vi "Main.vi"() -> ()   [LabVIEW 2015] (continued)
        n125 = call <vilib>:"Check if File or Folder Exists.vi"("error in (no error)"=w361, "path"=w363) -> ("error out"=w365:errorcluster, "file or folder exists?"=w364:bool, "dup path"=w366:path)  [unwired: 7 in]
        n126 = case shown="False" w364 {
          tunnel: w365 -> [w370 w371]
          tunnel: [w369 w371] -> w356
          tunnel: [w368 w372] -> w351
          tunnel: w366 -> [w367 w372]
          frame False {
            n127 = Create Folder(path (use dialog)=w367, error in=w370) -> (created path=w368:path, error out=w369:errorcluster)  [unwired: 1 in, 1 out]
          }
          frame True {
          }
        }
        n128 = property on="Calibration AI  Signals (Integrated)" class="WFChart (strict)"() -> ("History Data"=w358:dbl[][])  [unwired: 2 in, 2 out]
        n129 = Index Array(array=w337, index=2) -> (element=w347:cluster{"X":dbl[], "Y":dbl[]})
        n130 = Index Array(array=w337, index=3) -> (element=w346:cluster{"X":dbl[], "Y":dbl[]})
        n131 = Index Array(array=w337, index=0) -> (element=w349:cluster{"X":dbl[], "Y":dbl[]})
        n132 = Index Array(array=w337, index=1) -> (element=w348:cluster{"X":dbl[], "Y":dbl[]})
        n133 = Unbundle By Name(w346) -> ("Y"=w341:dbl[])
        n134 = Unbundle(w349) -> ("X"=w345:dbl[], "Y"=w344:dbl[])
        n135 = Unbundle By Name(w348) -> ("Y"=w343:dbl[])
        n136 = Unbundle By Name(w347) -> ("Y"=w342:dbl[])
        n137 = Transpose 2D Array(2D array=w358) -> (transposed array=w357:dbl[][])
        n138 = Build Array(w345, w344, w343, w342, w341) -> (w340:dbl[][])
        n139 = Transpose 2D Array(2D array=w340) -> (transposed array=w339:dbl[][])
        n140 = call "Save2CSV.vi"("Time Stamp?"=FALSE, "File Name"=w329, "error in"=w356, "Data Name"="Raw" ("string"), "Data 2D Array"=w357, "Parent Directory"=w351) -> ("error out"=w352:errorcluster)  [unwired: 4 in, 1 out]
        n141 = call "Save2CSV.vi"("Time Stamp?"=FALSE, "File Name"=w329, "error in"=w352, "Data Name"="Phase" ("string"), "Data 2D Array"=w339, "Parent Directory"=w351) -> ("error out"=w338:errorcluster)  [unwired: 4 in, 1 out]
      }
      event "Save #1": Value Change {
        n142 = event-data() -> ()  [unwired: 1 in, 1 out]
        n143 = local read "Wavelength (nm)"() -> (w380:string)
        n144 = local write "Wavelength #1"(w380) -> ()
        "[M/B]#1" <- "[M/B]"
        "Calibrated Bias #1" <- "Calibrated Bias (V)"
        "[O_B] #1" <- "[O_B]"
        "[d13]#1" <- "[d13]"
        "[d24]#1" <- "[d24]"
      }
      event "Load #1": Value Change {
        n145 = event-data() -> ()  [unwired: 1 in, 1 out]
        n146 = local read "[O_B] #1"() -> (w388:dbl)
        n147 = local read "[d13]#1"() -> (w384:dbl)
        n148 = local read "[d24]#1"() -> (w383:dbl)
        n149 = local read "Calibrated Bias #1"() -> (w390:dbl[])
        n150 = local read "[M/B]#1"() -> (w389:dbl)
        n151 = local write "[O_B]"(w388) -> ()
        n152 = local write "Calibrated Bias (V)"(w390) -> ()
        n153 = local write "Wavelength (nm)"("Wavelength #1") -> ()
        n154 = local write "[M/B]"(w389) -> ()
        n155 = local write "[d13]"(w384) -> ()
        n156 = local write "[d24]"(w383) -> ()
      }
      event "Save #2": Value Change {
        n157 = event-data() -> ()  [unwired: 1 in, 1 out]
        n158 = local read "[d13]"() -> (→"[d13]#2":dbl)
        n159 = local read "[O_B]"() -> (→"[O_B]#2":dbl)
        n160 = local read "[d24]"() -> (→"[d24]#2":dbl)
        n161 = local read "Calibrated Bias (V)"() -> (→"Calibrated Bias #2":dbl[])
        n162 = local read "Wavelength (nm)"() -> (w397:string)
        n163 = local read "[M/B]"() -> (→"[M/B]#2":dbl)
        n164 = local write "Wavelength #2"(w397) -> ()
      }
      event "Load #2": Value Change {
        n165 = event-data() -> ()  [unwired: 1 in, 1 out]
        n166 = local read "[O_B]#2"() -> (w408:dbl)
        n167 = local read "[d13]#2"() -> (w404:dbl)
        n168 = local read "Calibrated Bias #2"() -> (w412:dbl[])
        n169 = local read "[d24]#2"() -> (w403:dbl)
        n170 = local read "[M/B]#2"() -> (w411:dbl)
        n171 = local write "[O_B]"(w408) -> ()
        n172 = local write "Wavelength (nm)"("Wavelength #2") -> ()
        n173 = local write "Calibrated Bias (V)"(w412) -> ()
        n174 = local write "[M/B]"(w411) -> ()
        n175 = local write "[d24]"(w403) -> ()
        n176 = local write "[d13]"(w404) -> ()
      }
      event "Save #3": Value Change {
        n177 = event-data() -> ()  [unwired: 1 in, 1 out]
        n178 = local read "[O_B]"() -> (→"[O_B]#3":dbl)
        n179 = local read "[d24]"() -> (→"[d24]#3":dbl)
        n180 = local read "[d13]"() -> (→"[d13]#3":dbl)
        n181 = local read "Calibrated Bias (V)"() -> (→"Calibrated Bias #3":dbl[])
        n182 = local read "Wavelength (nm)"() -> (w417:string)
        n183 = local read "[M/B]"() -> (→"[M/B]#3":dbl)
        n184 = local write "Wavelength #3"(w417) -> ()
      }
      event "Load #3": Value Change {
        n185 = event-data() -> ()  [unwired: 1 in, 1 out]
        n186 = local read "[O_B]#3"() -> (w428:dbl)
        n187 = local read "[d13]#3"() -> (w424:dbl)
        n188 = local read "[d24]#3"() -> (w423:dbl)
        n189 = local read "Calibrated Bias #3"() -> (w430:dbl[])
        n190 = local read "[M/B]#3"() -> (w429:dbl)
        n191 = local write "[O_B]"(w428) -> ()
        n192 = local write "Wavelength (nm)"("Wavelength #3") -> ()
        n193 = local write "Calibrated Bias (V)"(w430) -> ()
        n194 = local write "[M/B]"(w429) -> ()
        n195 = local write "[d13]"(w424) -> ()
        n196 = local write "[d24]"(w423) -> ()
      }
      event "Save #4": Value Change {
        n197 = event-data() -> ()  [unwired: 1 in, 1 out]
        n198 = local read "[d13]"() -> (→"[d13]#4":dbl)
        n199 = local read "[d24]"() -> (→"[d24]#4":dbl)
        n200 = local read "[O_B]"() -> (→"[O_B]#4":dbl)
        n201 = local read "Calibrated Bias (V)"() -> (→"Calibrated Bias #4":dbl[])
        n202 = local read "Wavelength (nm)"() -> (w437:string)
        n203 = local read "[M/B]"() -> (→"[M/B]#4":dbl)
        n204 = local write "Wavelength #4"(w437) -> ()
      }
      event "Load #4": Value Change {
        n205 = event-data() -> ()  [unwired: 1 in, 1 out]
        n206 = local read "[O_B]#4"() -> (w448:dbl)
        n207 = local read "[d13]#4"() -> (w444:dbl)
        n208 = local read "Calibrated Bias #4"() -> (w450:dbl[])
        n209 = local read "[d24]#4"() -> (w443:dbl)
        n210 = local read "[M/B]#4"() -> (w449:dbl)
        n211 = local write "[O_B]"(w448) -> ()
        n212 = local write "Wavelength (nm)"("Wavelength #4") -> ()
        n213 = local write "Calibrated Bias (V)"(w450) -> ()
        n214 = local write "[M/B]"(w449) -> ()
        n215 = local write "[d13]"(w444) -> ()
        n216 = local write "[d24]"(w443) -> ()
      }
      event "Fast Scan": Value Change {
        # "Repeat for Fast Scan"
        n217 = event-data() -> ()  [unwired: 1 in, 1 out]
        n218 = flat-sequence {
          tunnel: w469 -> [w476]
          tunnel: [w476] -> w465
          tunnel: [w475] -> w464
          tunnel: [w474] -> w463
          tunnel: w467 -> [w474]
          tunnel: [w473] -> w462
          tunnel: w466 -> [w473]
          tunnel: w461 -> [w471]
          tunnel: [w470] -> w460
          tunnel: w465 -> [w502]
          tunnel: [w502] -> w457
          tunnel: w464 -> [w501]
          tunnel: [w501] -> w456
          tunnel: w463 -> [w497]
          tunnel: w462 -> [w484]
          tunnel: [w494] -> w455
          tunnel: w460 -> [w493]
          tunnel: [w482] -> w453
          tunnel: [w529] -> w459
          tunnel: [w530] -> w468
          tunnel: w457 -> [w530]
          tunnel: w455 -> [w526]
          tunnel: w456 -> [w520]
          tunnel: w453 -> [w513]
          frame #0 {
            n219 = local read "Shutter"() -> (w472:bool)
            n220 = case shown="False" w472 {
              tunnel: w471 -> [w479 w481]
              tunnel: [w478 w481] -> w470
              frame False {
                n221 = call "ShutterControl.vi"("error in"=w479, "Shutter"=TRUE) -> ("error out"=w478:errorcluster, "Status Indicator"=w477:bool)  [unwired: 8 in]
                n222 = local write "Shutter"(w477) -> ()
              }
              frame True {
              }
            }
            n223 = Tick Count (ms)() -> (millisecond timer value=w475:u32)
          }
          frame #1 {
            w487 = T13."Fast Scan" ("Main Tab")
            n224 = call "DAQInit.vi"("Scan/Meas Parameters"="Fast Scan Parameters", "error in"=w493, "Functions"=w487, "Global Parameters"=w484, "DAQ Channels"=w497) -> ("error out"=w495:errorcluster, "Expected Time (s)"=→"Expected Frame Time (s)":dbl, "Tasks Out"=w499:T14)  [unwired: 4 in]
            n225 = call "ScanXY.vi"("Scan/Meas Parameters"="Fast Scan Parameters") -> ("XYcoordinates"=w488:dbl[][])  [unwired: 10 in]
            n226 = Unbundle By Name("Fast Scan Parameters") -> ("Pixel Size"=w492:dbl)
            n227 = case shown="True" "Single Pixel?" {
              tunnel: [w503 w504] -> w489
              tunnel: w488 -> [w503 w505]
              frame False {
              }
              frame True {
                n228 = Multiply(x=w505, y=0.0) -> (x*y=w504:dbl[][])
              }
            }
            n229 = To Long Integer(number=w492) -> (32bit integer=w491:i32)
            n230 = call "ImageFrame.vi"("Tasks In"=w499, "Functions"=w487, "error in"=w495, "XYcoordinates"=w489) -> ("Tasks Out"=w496:T14, "DC AI Channel Date"=w485:dbl[], "error out"=w498:errorcluster)  [unwired: 7 in, 2 out]
            n231 = call "Analysis.vi"("Functions"=w487, "Scan/Meas Parameters"="Fast Scan Parameters", "Global Parameters"=w484, "DC AI Channel Data"=w485) -> ("AI DC Data"=w482:dbl[])  [unwired: 2 in, 5 out]
            n232 = Reshape Array(w482, w491, w491) -> (→"Fast Scan Intensity Image":dbl[][])
            n233 = call "DAQClose.vi"("error in"=w498, "Functions"=w487, "Tasks In"=w496, "DAQ Channels"=w497) -> ("error out"=w494:errorcluster)  [unwired: 7 in]
          }
          frame #2 {
            n234 = local read "Simple Max Search"() -> (w516:bool)
            n235 = local read "Export Z Calibration"() -> (w507:bool)
            n236 = Tick Count (ms)() -> (millisecond timer value=w521:u32)
            n237 = call "ShutterControl.vi"("error in"=w526, "Shutter"=FALSE) -> ("error out"=w525:errorcluster, "Status Indicator"=w527:bool)  [unwired: 8 in]
            n238 = local read "Quadratic Search"() -> (w509:bool)
            n239 = local write "Shutter"(w527) -> ()
            n240 = call <vilib>:"Std Deviation and Variance.vi"("X"=w513) -> ("mean"=w508:dbl, "variance"=w514:dbl)  [unwired: 1 in, 1 out]
            "Mean Pixel Value" <- w508
            n241 = Subtract(x=w521, y=w520) -> (x-y=w523:u32)
            n242 = Square(x=w508) -> (x^2=w515:dbl)
            n243 = local read "SPGD"() -> (w517:bool)
            n244 = To Double Precision Float(number=w523) -> (double precision float=w524:dbl)
            n245 = Divide(x=w514, y=w515) -> (x/y=w510:dbl)
            "Normalized Variance" <- w510
            n246 = Divide(x=w524, y=1000.0) -> (x/y=→"Actual Scan Time (s)":dbl)
            n247 = Compound Arithmetic op=OR(w509, w517, w516, w507) -> (w518:bool)
            n248 = case shown="False" w518 {
              tunnel: [w546 w553] -> w529
              tunnel: w525 -> [w544 w553]
              frame False {
                n249 = local read "Fast Scan Progress"() -> (w540:dbl)
                n250 = Reciprocal(x="Fast Scan Frames") -> (1/x=w541:dbl)
                n251 = Multiply(x=100.0, y=w541) -> (x*y=w543:dbl)
                n252 = Add(x=w540, y=w543) -> (x+y=w536:dbl)
                "Fast Scan Progress" <- w536
                n253 = Greater Or Equal?(x=w536, y=100.0) -> (x >= y?=w537:bool)
                n254 = Compound Arithmetic op=OR(w537, "Stop Fast Scan") -> (w545:bool)
                n255 = case shown="True" w545 {
                  tunnel: w544 -> [w549 w550]
                  tunnel: [w548 w550] -> w546
                  frame False {
                    # "Continue Fast Scan"
                    n256 = property on="Fast Scan" class="Bool (strict)"(error in=w549, "Val(Sgnl)"=TRUE ("Value (Signaling)")) -> (error out=w548:errorcluster)  [unwired: 1 in, 1 out]
                  }
                  frame True {
                    w552 = FALSE ("Fast Scan")
                    # "Fast Scan Stops"
                    n257 = local write "Fast Scan Progress"(0.0 ("Fast Scan Progress")) -> ()
                    n258 = local write "Fast Scan"(w552) -> ()
                    n259 = local write "Stop Fast Scan"(w552) -> ()
                  }
                }
              }
              frame True {
              }
            }
            n260 = case shown="\"Mean Squared Pixel Value\"" "Optimization Metric" {
              tunnel: [w531 w532 w533] -> w511
              tunnel: w508 -> [w531 _ w534]
              tunnel: w510 -> [_ w532 _]
              frame "Mean Pixel Value", Default {
              }
              frame "Normalized Variance" {
              }
              frame "Mean Squared Pixel Value" {
                n261 = Square Root(x=w534) -> (sqrt(x)=w533:dbl)
              }
            }
            "Metric Value" <- w511
          }
        }
      }
      event "Relax DM": Value Change {
        w566 = u32 0 items=["Mirror", "Arms", "Mirror + Arms"] ("Device Part (Mirror)")
        # "First Step"
        n262 = event-data() -> ()  [unwired: 1 in, 1 out]
        n263 = call "TLDFMX Relax.vi"("Reload (1)"=TRUE, "error in (no error)"=w554, "Is First Step (0)"=TRUE, "Device Part (Mirror)"=w566, "instrument handle"=w555) -> ("error out"=w562:errorcluster, "Relax Pattern Mirror (0)"=w561:dbl[], "instrument handle out"=w563:refnum<visa-resource-name>)  [unwired: 2 in, 2 out]
        n264 = call "TLDFM Set Segment Voltages.vi"("error in (no error)"=w562, "Segment Voltages"=w561, "instrument handle"=w563) -> ("error out"=w559:errorcluster, "instrument handle out"=w560:refnum<visa-resource-name>)  [unwired: 7 in]
        n265 = while {
          tunnel: w560 -> [w573]
          tunnel: w559 -> [w572]
          tunnel: [w569] -> w558
          tunnel: [w568] -> w557
          stop <- w570 stop-if-true
          w574 = u32 0 items=["Mirror", "Arms", "Mirror + Arms"] ("Device Part (Mirror)")
          # "Loop Until Remaining Relax Steps Are 0"
          n266 = call "TLDFMX Relax.vi"("Reload (1)"=TRUE, "error in (no error)"=w572, "Is First Step (0)"=FALSE, "Device Part (Mirror)"=w574, "instrument handle"=w573) -> ("error out"=w578:errorcluster, "Relax Pattern Mirror (0)"=w579:dbl[], "instrument handle out"=w577:refnum<visa-resource-name>, "Remaining Steps"=w571:i32)  [unwired: 2 in, 1 out]
          n267 = Less Or Equal To 0?(x=w571) -> (x <= 0?=w570:bool)
          n268 = call "TLDFM Set Segment Voltages.vi"("error in (no error)"=w578, "Segment Voltages"=w579, "instrument handle"=w577) -> ("error out"=w568:errorcluster, "instrument handle out"=w569:refnum<visa-resource-name>)  [unwired: 7 in]
        }
      }
      event "Reset Zernike": Value Change {
        n269 = event-data() -> ()  [unwired: 1 in, 1 out]
        n270 = call "TLDFMX Reset.vi"("error in (no error)"=w582, "instrument handle"=w583) -> ("error out"=w580:errorcluster, "instrument handle out"=w581:refnum<visa-resource-name>)  [unwired: 8 in]
        n271 = local write "Zernike Array"(dbl[] [0.0, 0.0, 0.0, 0.0, 0.0, 0.0, 0.0, 0.0, 0.0, 0.0, 0.0, 0.0] ("Zernike Array")) -> ()
      }
      event "Zernike Array", "Apply Zernike": Value Change {
        n272 = event-data() -> ()  [unwired: 1 in, 1 out]
        n273 = local read "Zernike Enable"() -> (w589:bool[])
        n274 = Boolean To (0,1)(Boolean=w589) -> (0, 1=w588:i16[])
        n275 = Multiply(x="Zernike Array", y=w588) -> (x*y=w586:dbl[])
        n276 = call "TLDFMX Calculate Zernike Pattern.vi"("error in (no error)"=w599, "Zernike Amplitudes"=w586, "Zernikes"=u32 4294967295, "instrument handle"=w597) -> ("error out"=w594:errorcluster, "Mirror Pattern"=w595:dbl[], "instrument handle out"=w596:refnum<visa-resource-name>)  [unwired: 5 in]
        n277 = call "TLDFM Set Segment Voltages.vi"("error in (no error)"=w594, "Segment Voltages"=w595, "instrument handle"=w596) -> ("error out"=w593:errorcluster, "instrument handle out"=w591:refnum<visa-resource-name>)  [unwired: 7 in]
      }
      event "Save Zernike": Value Change {
        w617 = "DM" ("section")
        n278 = event-data() -> ()  [unwired: 1 in, 1 out]
        n279 = Current VI's Path() -> (path=w601:path)
        n280 = Strip Path(path=w601) -> (stripped path=w600:path)  [unwired: 1 out]
        n281 = Build Path(base path=w600, name or relative path=path "config.ini" ("default name")) -> (appended path=w627:path)
        n282 = local read "Zernike Array"() -> (w611:dbl[])
        n283 = call <vilib>:"Open Config Data.vi"("error in (no error)"=w626, "create file if necessary (T)"=TRUE, "configuration file path"=w627) -> ("error out"=w625:errorcluster, "refnum"=w623:T15)  [unwired: 6 in, 1 out]
        n284 = Array To Spreadsheet String(delimiter (Tab)=",", array=w611, 3:"%#g" ("format string")) -> (spreadsheet string=w615:string)
        n285 = Search and Replace String(input string=w615, search string="\r\n") -> (result string=w610:string)  [unwired: 6 in, 3 out]
        n286 = call-poly <vilib>:"Write Key.vi"("section"=w617, "error in (no error)"=w625, "value"=w610, "key"="Zernike Array", "refnum"=w623) -> ("error out"=w619:errorcluster, "refnum out"=w621:T15)  [unwired: 4 in, 1 out]
        n287 = local read "Zernike Enable"() -> (w604:bool[])
        n288 = for {
          tunnel: w604 -> [w632] mode=indexing
          tunnel: [w631] -> w605 mode=indexing
          n289 = Select(t="TRUE", s=w632, f="FALSE") -> (s? t:f=w631:string)
        }
        n290 = Array To Spreadsheet String(delimiter (Tab)=",", array=w605, 3:"%s" ("format string")) -> (spreadsheet string=w609:string)
        n291 = Search and Replace String(input string=w609, search string="\r\n") -> (result string=w603:string)  [unwired: 6 in, 3 out]
        n292 = call-poly <vilib>:"Write Key.vi"("section"=w617, "error in (no error)"=w619, "value"=w603, "key"="Zernike Enable", "refnum"=w621) -> ("error out"=w618:errorcluster, "refnum out"=w620:T15)  [unwired: 4 in, 1 out]
        n293 = call <vilib>:"Close Config Data.vi"("error in (no error)"=w618, "refnum"=w620) -> ("error out"=w624:errorcluster)  [unwired: 8 in, 1 out]
      }
      event "Load Zernike": Value Change {
        n294 = event-data() -> ()  [unwired: 1 in, 1 out]
        n295 = Current VI's Path() -> (path=w642:path)
        n296 = Strip Path(path=w642) -> (stripped path=w641:path)  [unwired: 1 out]
        n297 = Build Path(base path=w641, name or relative path=path "config.ini" ("default name")) -> (appended path=w639:path)
        n298 = call <vilib>:"Check if File or Folder Exists.vi"("error in (no error)"=w638, "path"=w639) -> ("error out"=w637:errorcluster, "file or folder exists?"=w635:bool, "dup path"=w636:path)  [unwired: 7 in]
        n299 = case shown="True" w635 {
          tunnel: [w646 w670] -> w640
          tunnel: w637 -> [w646 w648]
          tunnel: w636 -> [_ w647]
          frame False {
          }
          frame True {
            w650 = "DM" ("section")
            n300 = call <vilib>:"Open Config Data.vi"("error in (no error)"=w648, "create file if necessary (T)"=FALSE, "configuration file path"=w647) -> ("error out"=w663:errorcluster, "refnum"=w664:T15)  [unwired: 6 in, 1 out]
            n301 = call-poly <vilib>:"Read Key.vi"("section"=w650, "error in (no error)"=w663, "key"="Zernike Array", "refnum"=w664) -> ("error out"=w655:errorcluster, "value"=w666:string, "refnum out"=w653:T15)  [unwired: 4 in, 1 out]
            n302 = Spreadsheet String To Array(delimiter (Tab)=",", format string="%s", spreadsheet string=w666, array type (2D Dbl)=dbl[] []) -> (array=w662:dbl[])
            n303 = local write "Zernike Array"(w662) -> ()
            n304 = call-poly <vilib>:"Read Key.vi"("section"=w650, "error in (no error)"=w655, "key"="Zernike Enable", "refnum"=w653) -> ("error out"=w654:errorcluster, "value"=w658:string, "refnum out"=w652:T15)  [unwired: 4 in, 1 out]
            n305 = Spreadsheet String To Array(delimiter (Tab)=",", format string="%s", spreadsheet string=w658, array type (2D Dbl)=string[] []) -> (array=w656:string[])
            n306 = for {
              tunnel: "TRUE" -> [w674]
              tunnel: w656 -> [w673] mode=indexing
              tunnel: [w672] -> w649 mode=indexing
              n307 = Equal?(x=w673, y=w674) -> (x = y?=w672:bool)
            }
            n308 = local write "Zernike Enable"(w649) -> ()
            n309 = call <vilib>:"Close Config Data.vi"("error in (no error)"=w654, "refnum"=w652) -> ("error out"=w670:errorcluster)  [unwired: 8 in, 1 out]
          }
        }
      }
      event "Quadratic Search": Value Change {
        n310 = event-data() -> ()  [unwired: 1 in, 1 out]
        n311 = while {
          tunnel: [w776] -> w682
          tunnel: [w778] -> w686
          stop <- w779 stop-if-true
          n312 = local read "Zernike Enable"() -> (w777:bool[])
          n313 = local read "Current Z Idx"() -> (w782:i32)
          n314 = Index Array(array=w777, index=w782) -> (element=w783:bool)
          n315 = Array Size(array=w777) -> (size(s)=w781:i32)
          n316 = case shown="True" w783 {
            tunnel: w782 -> [w787 w789]
            tunnel: [w786 w789] -> w776
            tunnel: [FALSE ("2D Time-Lapse Measure") TRUE ("2D Time-Lapse Measure")] -> w780
            frame False {
              n317 = local write "Z Direction"(TRUE ("Zernike Dir")) -> ()
              n318 = Increment(x=w787) -> (x+1=w786:i32)
            }
            frame True {
            }
          }
          n319 = Greater?(x=w776, y=w781) -> (0:w778:bool)
          n320 = local write "Current Z Idx"(w776) -> ()
          n321 = Compound Arithmetic op=OR(w780, w778) -> (w779:bool)
        }
        n322 = local read "Current Iteration"() -> (w675:sgl)
        n323 = local read "Quadratic Calc"() -> (w678:bool)
        n324 = case shown="False" w678 {
          tunnel: w677 -> [w689 w693]
          tunnel: [w689 w693] -> w676
          tunnel: w675 -> [w688 _]
          frame False {
            n325 = Equal To 0?(x=w688) -> (x = 0?=w687:bool)
            n326 = case shown="True" w687 {
              frame False {
              }
              frame True {
                n327 = local read "Zernike Array"() -> (w690:dbl[])
                n328 = local write "Optimal Z Idx"(0 ("Optimal Z Idx")) -> ()
                n329 = local write "Optimal Zernike"(w690) -> ()
              }
            }
          }
          frame True {
            n330 = local read "Bias Amplitude"() -> (w702:dbl)
            n331 = local read "Optimal Zernike"() -> (w696:dbl[])
            n332 = local read "Initial Metric"() -> (w704:dbl)
            n333 = local read "Metric Value"() -> (w703:dbl)
            n334 = local read "Last Metric"() -> (w705:dbl)
            n335 = local read "Optimal Z Idx"() -> (w692:i32)
            n336 = call "QuadraticOptimization.vi"("Bias Amplitude"=w702, "Neg Metric"=w703, "Initial Metric"=w704, "Pos Metric"=w705) -> ("Opt Variable (compared to 0)"=w694:dbl)  [unwired: 7 in]
            n337 = Index Array(array=w696, index=w692) -> (element=w698:dbl)
            n338 = Add(x=w698, y=w694) -> (x+y=w699:dbl)
            n339 = In Range and Coerce(upper limit=1.0 ("y"), x=w699, lower limit=-1.0 ("y")) -> (coerced(x)=w697:dbl)  [unwired: 1 out]
            n340 = Replace Array Subset(array=w696, new element=w697, index=w692) -> (→"Optimal Zernike":dbl[])
          }
        }
        n341 = local read "Stop AO Algorithm"() -> (w685:bool)
        n342 = Compound Arithmetic op=OR(w686, w685) -> (w684:bool)
        n343 = case shown="False" w684 {
          tunnel: w676 -> [w717 w765]
          tunnel: [w712 w764] -> w683
          tunnel: w680 -> [w718 w762]
          tunnel: [w719 w763] -> w679
          tunnel: w675 -> [w709 _]
          tunnel: w682 -> [w714 _]
          frame False {
            w711 = TRUE ("Value (Signaling)")
            n344 = Equal To 0?(x=w709) -> (x = 0?=w715:bool)
            n345 = case shown="False" w715 {
              tunnel: [w738 w755] -> w710
              tunnel: [w740 w756] -> w706
              tunnel: w714 -> [w726 _]
              frame False {
                n346 = local read "Initial Zernike"() -> (w727:dbl[])
                n347 = local read "Z Direction"() -> (w737:bool)
                n348 = case shown="False" w737 {
                  tunnel: "Bias Amplitude" -> [w748 w753]
                  tunnel: [w747 w753] -> w735
                  tunnel: [FALSE ("Zernike Dir") TRUE ("Zernike Dir")] -> w730
                  tunnel: w726 -> [w744 _]
                  frame False {
                    # "Negative Bias"
                    n349 = Multiply(x=w748, y=-1.0) -> (x*y=w747:dbl)
                    "Quadratic Calc" <- TRUE ("Quadratic Calc")
                    "Optimal Z Idx" <- w744
                  }
                  frame True {
                    # "Positive Bias"
                    n350 = local write "Quadratic Calc"(FALSE ("Zernike Dir")) -> ()
                    n351 = local write "Z Direction"(FALSE ("Zernike Dir")) -> ()
                  }
                }
                n352 = Index Array(array=w727, index=w726) -> (element=w739:dbl)
                n353 = Add(x=w739, y=w735) -> (x+y=w732:dbl)
                n354 = In Range and Coerce(upper limit=1.0 ("y"), x=w732, lower limit=-1.0 ("y")) -> (coerced(x)=w731:dbl, In Range?=w729:bool)
                n355 = Compound Arithmetic op=AND(w729, w730) -> (w728:bool)
                n356 = case shown="False" w728 {
                  tunnel: w726 -> [w742 _]
                  frame False {
                    n357 = Increment(x=w742) -> (x+1=w743:i32)
                    n358 = local write "Z Direction"(TRUE ("Zernike Dir")) -> ()
                    n359 = local write "Current Z Idx"(w743) -> ()
                  }
                  frame True {
                  }
                }
                n360 = local read "Metric Value"() -> (w740:dbl)
                n361 = Replace Array Subset(array=w727, new element=w731, index=w726) -> (w738:dbl[])
              }
              frame True {
                n362 = local read "Zernike Array"() -> (w755:dbl[])
                "Initial Zernike" <- w755
                n363 = local read "Last Metric"() -> (w756:dbl)
                n364 = local write "Quadratic Calc"(FALSE ("Zernike Dir")) -> ()
              }
            }
            n365 = Increment(x=w709) -> (x+1=w716:sgl)
            n366 = local write "Current Iteration"(w716) -> ()
            n367 = call "TLDFMX Calculate Zernike Pattern.vi"("error in (no error)"=w717, "Zernike Amplitudes"=w710, "Zernikes"=u32 4294967295, "instrument handle"=w718) -> ("error out"=w721:errorcluster, "Mirror Pattern"=w722:dbl[], "instrument handle out"=w723:refnum<visa-resource-name>)  [unwired: 5 in]
            n368 = call "TLDFM Set Segment Voltages.vi"("error in (no error)"=w721, "Segment Voltages"=w722, "instrument handle"=w723) -> ("error out"=w720:errorcluster, "instrument handle out"=w719:refnum<visa-resource-name>)  [unwired: 7 in]
            n369 = Equal?(x=w709, y=sgl 1.0) -> (x = y?=w707:bool)
            n370 = property on="Fast Scan" class="Bool (strict)"(error in=w720, "Val(Sgnl)"=w711) -> (error out=w713:errorcluster)  [unwired: 1 in, 1 out]
            n371 = case shown="True" w707 {
              tunnel: w706 -> [_ w725]
              frame False {
              }
              frame True {
                "Initial Metric" <- w725
              }
            }
            n372 = local write "Zernike Array"(w710) -> ()
            n373 = property on="Quadratic Search" class="Bool (strict)"(error in=w713, "Val(Sgnl)"=w711) -> (error out=w712:errorcluster)  [unwired: 1 in, 1 out]
            n374 = local write "Last Metric"(w706) -> ()
          }
          frame True {
            w775 = FALSE ("2D Time-Lapse Measure")
            n375 = local read "Zernike Enable"() -> (w761:bool[])
            n376 = local read "Optimal Zernike"() -> (w759:dbl[])
            n377 = Boolean To (0,1)(Boolean=w761) -> (0, 1=w760:i16[])
            n378 = Multiply(x=w759, y=w760) -> (x*y=w758:dbl[])
            n379 = call "TLDFMX Calculate Zernike Pattern.vi"("error in (no error)"=w765, "Zernike Amplitudes"=w758, "Zernikes"=u32 4294967295, "instrument handle"=w762) -> ("error out"=w766:errorcluster, "Mirror Pattern"=w767:dbl[], "instrument handle out"=w768:refnum<visa-resource-name>)  [unwired: 5 in]
            n380 = local write "Zernike Array"(w759) -> ()
            n381 = call "TLDFM Set Segment Voltages.vi"("error in (no error)"=w766, "Segment Voltages"=w767, "instrument handle"=w768) -> ("error out"=w764:errorcluster, "instrument handle out"=w763:refnum<visa-resource-name>)  [unwired: 7 in]
            n382 = local write "Quadratic Calc"(FALSE ("Zernike Dir")) -> ()
            n383 = local write "Optimal Z Idx"(0 ("Optimal Z Idx")) -> ()
            n384 = local write "Current Iteration"(sgl 0.0 ("Current Step")) -> ()
            n385 = local write "Quadratic Search"(w775) -> ()
            n386 = local write "Z Direction"(TRUE ("Zernike Dir")) -> ()
            n387 = local write "Fast Scan Progress"(0.0 ("Fast Scan Progress")) -> ()
            n388 = local write "Current Z Idx"(0 ("Curr Zernike Idx")) -> ()
            n389 = local write "Fast Scan"(w775) -> ()
            n390 = local write "Stop Fast Scan"(w775) -> ()
            n391 = local write "Stop AO Algorithm"(w775) -> ()
          }
        }
      }
      event "Simple Max Search": Value Change {
        n392 = event-data() -> ()  [unwired: 1 in, 1 out]
        n393 = while {
          tunnel: [w800] -> w790
          tunnel: [w802] -> w792
          stop <- w803 stop-if-true
          n394 = local read "Zernike Enable"() -> (w801:bool[])
          n395 = local read "Current Z Idx"() -> (w806:i32)
          n396 = Index Array(array=w801, index=w806) -> (element=w807:bool)
          n397 = Array Size(array=w801) -> (size(s)=w805:i32)
          n398 = case shown="False" w807 {
            tunnel: w806 -> [w811 w813]
            tunnel: [w810 w813] -> w800
            tunnel: [FALSE ("2D Time-Lapse Measure") TRUE ("2D Time-Lapse Measure")] -> w804
            frame False {
              n399 = local write "Z Direction"(TRUE ("Zernike Dir")) -> ()
              n400 = Increment(x=w811) -> (x+1=w810:i32)
            }
            frame True {
            }
          }
          n401 = Greater?(x=w800, y=w805) -> (0:w802:bool)
          n402 = local write "Current Z Idx"(w800) -> ()
          n403 = Compound Arithmetic op=OR(w804, w802) -> (w803:bool)
        }
        n404 = local read "Stop AO Algorithm"() -> (w794:bool)
        n405 = local read "Current Iteration"() -> (w791:sgl)
        n406 = Compound Arithmetic op=OR(w792, w794) -> (w793:bool)
        n407 = case shown="False" w793 {
          tunnel: w798 -> [w814 w871]
          tunnel: w797 -> [w815 w872]
          tunnel: [w829 w872] -> w796
          tunnel: [w826 w871] -> w795
          tunnel: w791 -> [w818 _]
          tunnel: w790 -> [w819 _]
          frame False {
            w825 = TRUE ("Value (Signaling)")
            n408 = Equal To 0?(x=w818) -> (x = 0?=w824:bool)
            n409 = Increment(x=w818) -> (x+1=w817:sgl)
            n410 = case shown="True" w824 {
              tunnel: [w841 w867] -> w821
              tunnel: w819 -> [w836 _]
              tunnel: [w834 w866] -> w816
              frame False {
                n411 = local read "Metric Value"() -> (w834:dbl)
                n412 = local read "Zernike Array"() -> (w843:dbl[])
                n413 = local read "Last Metric"() -> (w835:dbl)
                n414 = local read "Z Direction"() -> (w837:bool)
                n415 = Greater?(x=w834, y=w835) -> (0:w840:bool)
                n416 = Index Array(array=w843, index=w836) -> (element=w844:dbl)
                n417 = case shown="True" w837 {
                  tunnel: w840 -> [w848 w859]
                  tunnel: "Step Size" -> [w847 w858]
                  tunnel: [w846 w857] -> w838
                  tunnel: w836 -> [w845 _]
                  frame False {
                    # "Decreasing Zernike Coefficient"
                    n418 = case shown="True" w848 {
                      tunnel: w847 -> [w852 w854]
                      tunnel: [w852 w853] -> w846
                      tunnel: w845 -> [w850 _]
                      frame False {
                        n419 = Increment(x=w850) -> (x+1=w851:i32)
                        n420 = local write "Z Direction"(TRUE ("Zernike Dir")) -> ()
                        n421 = local write "Current Z Idx"(w851) -> ()
                      }
                      frame True {
                        n422 = local write "Z Direction"(FALSE ("Zernike Dir")) -> ()
                        n423 = Multiply(x=w854, y=-1.0) -> (x*y=w853:dbl)
                      }
                    }
                  }
                  frame True {
                    # "Increasing Zernike Coefficient"
                    n424 = case shown="False" w859 {
                      tunnel: w858 -> [w863 w865]
                      tunnel: [w862 w865] -> w857
                      frame False {
                        n425 = local write "Z Direction"(FALSE ("Zernike Dir")) -> ()
                        n426 = Multiply(x=w863, y=-1.0) -> (x*y=w862:dbl)
                      }
                      frame True {
                        "Z Direction" <- TRUE ("Zernike Dir")
                      }
                    }
                  }
                }
                n427 = Add(x=w844, y=w838) -> (x+y=w842:dbl)
                n428 = Replace Array Subset(array=w843, new element=w842, index=w836) -> (w841:dbl[])
              }
              frame True {
                n429 = local read "Zernike Array"() -> (w867:dbl[])
                n430 = local read "Last Metric"() -> (w866:dbl)
              }
            }
            "Last Metric" <- w816
            n431 = local write "Current Iteration"(w817) -> ()
            n432 = In Range and Coerce(upper limit=1.0 ("y"), x=w821, lower limit=-1.0 ("y")) -> (coerced(x)=w820:dbl[])  [unwired: 1 out]
            n433 = call "TLDFMX Calculate Zernike Pattern.vi"("error in (no error)"=w814, "Zernike Amplitudes"=w820, "Zernikes"=u32 4294967295, "instrument handle"=w815) -> ("error out"=w830:errorcluster, "Mirror Pattern"=w831:dbl[], "instrument handle out"=w832:refnum<visa-resource-name>)  [unwired: 5 in]
            n434 = call "TLDFM Set Segment Voltages.vi"("error in (no error)"=w830, "Segment Voltages"=w831, "instrument handle"=w832) -> ("error out"=w828:errorcluster, "instrument handle out"=w829:refnum<visa-resource-name>)  [unwired: 7 in]
            n435 = property on="Fast Scan" class="Bool (strict)"(error in=w828, "Val(Sgnl)"=w825) -> (error out=w827:errorcluster)  [unwired: 1 in, 1 out]
            n436 = local write "Zernike Array"(w820) -> ()
            n437 = property on="Simple Max Search" class="Bool (strict)"(error in=w827, "Val(Sgnl)"=w825) -> (error out=w826:errorcluster)  [unwired: 1 in, 1 out]
          }
          frame True {
            w873 = FALSE ("2D Time-Lapse Measure")
            n438 = local write "Z Direction"(TRUE ("Zernike Dir")) -> ()
            n439 = local write "Simple Max Search"(w873) -> ()
            n440 = local write "Fast Scan Progress"(0.0 ("Fast Scan Progress")) -> ()
            n441 = local write "Current Iteration"(sgl 0.0 ("Current Step")) -> ()
            n442 = local write "Fast Scan"(w873) -> ()
            n443 = local write "Stop Fast Scan"(w873) -> ()
            n444 = local write "Stop AO Algorithm"(w873) -> ()
            "Current Z Idx" <- 0 ("Curr Zernike Idx")
          }
        }
      }
      event "SPGD": Value Change {
        n445 = event-data() -> ()  [unwired: 1 in, 1 out]
        n446 = local read "Current Iteration"() -> (w885:sgl)
        n447 = To Single Precision Float(number="Total Iteration") -> (single precision float=w877:sgl)
        n448 = Greater Or Equal?(x=w885, y=w877) -> (x >= y?=w883:bool)
        n449 = Compound Arithmetic op=OR(w883, "Stop AO Algorithm") -> (w884:bool)
        n450 = case shown="False" w884 {
          tunnel: w885 -> [w894 _]
          tunnel: w881 -> [w888 w945]
          tunnel: [w897 w945] -> w876
          tunnel: w880 -> [w889 w944]
          tunnel: [w906 w944] -> w879
          frame False {
            w899 = TRUE ("Value (Signaling)")
            n451 = Equal To 0?(x=w894) -> (x = 0?=w901:bool)
            n452 = Quotient & Remainder(x=w894, y=sgl 1.0) -> (x-y*floor(x/y)=w913:sgl)  [unwired: 1 out]
            n453 = local read "Metric Value"() -> (w887:dbl)
            n454 = local read "Zernike Array"() -> (w905:dbl[])
            n455 = Equal?(x=w913, y=sgl 0.5) -> (x = y?=w911:bool)
            n456 = Add(x=w894, y=sgl 0.5) -> (x+y=→"Current Iteration":sgl)
            n457 = case shown="False" w911 {
              tunnel: [w917 w930] -> w902
              tunnel: w905 -> [_ w929]
              tunnel: w901 -> [w916 _]
              tunnel: w887 -> [w915 w928]
              frame False {
                # "Before First Sub-Step"
                n458 = case shown="False" w916 {
                  tunnel: [w920 w927] -> w917
                  tunnel: w915 -> [w924 _]
                  frame False {
                    n459 = local read "Sigma"() -> (w925:dbl[])
                    n460 = local read "Last Metric"() -> (w918:dbl)
                    n461 = local read "Last Zernike"() -> (w919:dbl[])
                    n462 = Multiply(x="Learning Rate", y=w925) -> (x*y=w923:dbl[])
                    n463 = Subtract(x=w924, y=w918) -> (x-y=w922:dbl)
                    n464 = Multiply(x=w923, y=w922) -> (x*y=w921:dbl[])
                    n465 = Subtract(x=w919, y=w921) -> (x-y=w920:dbl[])
                  }
                  frame True {
                    n466 = local read "Zernike Array"() -> (w927:dbl[])
                  }
                }
              }
              frame True {
                # "Before Second Sub-Step"
                n467 = local write "Last Metric"(w928) -> ()
                n468 = Array Size(array=w929) -> (size(s)=w932:i32)
                n469 = for {
                  N: w932 -> [_]
                  tunnel: [w933] -> w931 mode=indexing
                  # "4 possibilities, [0, 4)"
                  n470 = Random Number (0-1)() -> (number: 0 to 1=w937:dbl)
                  n471 = Multiply(x=w937, y=4.0) -> (x*y=w935:dbl)
                  n472 = Round Toward -Infinity(1:w935) -> (0:w934:dbl)
                  n473 = case shown="3" w934 {
                    tunnel: [-0.05 ("y") -0.025 ("y") 0.025 ("y") 0.05 ("y")] -> w933
                    frame 0, Default {
                    }
                    frame 1 {
                    }
                    frame 2 {
                    }
                    frame 3 {
                    }
                  }
                }
                "Sigma" <- w931
                n474 = Add(x=w929, y=w931) -> (x+y=w930:dbl[])
                "Last Zernike" <- w929
              }
            }
            n475 = In Range and Coerce(upper limit=1.0 ("y"), x=w902, lower limit=-1.0 ("y")) -> (coerced(x)=w893:dbl[])  [unwired: 1 out]
            n476 = Boolean To (0,1)(Boolean="Zernike Enable") -> (0, 1=w891:i16[])
            n477 = Multiply(x=w893, y=w891) -> (x*y=w890:dbl[])
            n478 = call "TLDFMX Calculate Zernike Pattern.vi"("error in (no error)"=w888, "Zernike Amplitudes"=w890, "Zernikes"=u32 4294967295, "instrument handle"=w889) -> ("error out"=w907:errorcluster, "Mirror Pattern"=w908:dbl[], "instrument handle out"=w909:refnum<visa-resource-name>)  [unwired: 5 in]
            n479 = call "TLDFM Set Segment Voltages.vi"("error in (no error)"=w907, "Segment Voltages"=w908, "instrument handle"=w909) -> ("error out"=w898:errorcluster, "instrument handle out"=w906:refnum<visa-resource-name>)  [unwired: 7 in]
            n480 = property on="Fast Scan" class="Bool (strict)"(error in=w898, "Val(Sgnl)"=w899) -> (error out=w900:errorcluster)  [unwired: 1 in, 1 out]
            n481 = property on="SPGD" class="Bool (strict)"(error in=w900, "Val(Sgnl)"=w899) -> (error out=w897:errorcluster)  [unwired: 1 in, 1 out]
            n482 = local write "Zernike Array"(w890) -> ()
          }
          frame True {
            w942 = FALSE ("2D Time-Lapse Measure")
            n483 = local write "Fast Scan Progress"(0.0 ("Fast Scan Progress")) -> ()
            n484 = local write "Fast Scan"(w942) -> ()
            n485 = local write "Current Iteration"(sgl 0.0 ("Current Step")) -> ()
            n486 = local write "SPGD"(w942) -> ()
            n487 = local write "Stop Fast Scan"(w942) -> ()
            n488 = local write "Stop AO Algorithm"(w942) -> ()
          }
        }
      }
      event "Export Z Calibration": Value Change {
        n489 = event-data() -> ()  [unwired: 1 in, 1 out]
        n490 = local read "Z Direction"() -> (w953:bool)
        n491 = local read "Current Iteration"() -> (w951:sgl)
        n492 = Less Or Equal?(x=w951, y=sgl 1.0) -> (x <= y?=w952:bool)
        n493 = Compound Arithmetic op=OR(w953, w952) -> (w954:bool)
        n494 = case shown="False" w954 {
          tunnel: w955 -> [w968 w993]
          tunnel: [w967 w993] -> w948
          frame False {
            n495 = local read "Current Z Idx"() -> (w966:i32)
            n496 = Add(x=w966, y=3) -> (x+y=w985:i32)
            n497 = Number To Decimal String(number=w985) -> (decimal integer string=w986:string)  [unwired: 1 in]
            n498 = Current VI's Path() -> (path=w982:path)
            n499 = Concatenate Strings("Zernike Calibration_" ("string"), "Note") -> (w964:string)
            n500 = Strip Path(path=w982) -> (stripped path=w983:path)  [unwired: 1 out]
            n501 = Build Path(base path=w983, name or relative path=w964) -> (appended path=w976:path)
            n502 = call <vilib>:"Check if File or Folder Exists.vi"("error in (no error)"=w968, "path"=w976) -> ("error out"=w978:errorcluster, "file or folder exists?"=w979:bool, "dup path"=w977:path)  [unwired: 7 in]
            n503 = case shown="False" w979 {
              tunnel: w978 -> [w990 w991]
              tunnel: [w989 w991] -> w975
              tunnel: [w988 w992] -> w981
              tunnel: w977 -> [w987 w992]
              frame False {
                n504 = Create Folder(path (use dialog)=w987, error in=w990) -> (created path=w988:path, error out=w989:errorcluster)  [unwired: 1 in, 1 out]
              }
              frame True {
              }
            }
            n505 = property on="Metric Calibration" class="WFChart (strict)"(error in=w975) -> (error out=w972:errorcluster, "History Data"=w974:dbl[][])  [unwired: 1 in, 1 out]
            n506 = Transpose 2D Array(2D array=w974) -> (transposed array=w973:dbl[][])
            n507 = call "Save2CSV.vi"("Time Stamp?"=FALSE, "File Name"="Z" ("string"), "error in"=w972, "Data Name"=w986, "Data 2D Array"=w973, "Parent Directory"=w981) -> ("error out"=w969:errorcluster)  [unwired: 4 in, 1 out]
            n508 = property on="Metric Calibration" class="WFChart (strict)"(error in=w969, "History Data"=dbl[][] []) -> (error out=w967:errorcluster)  [unwired: 1 in, 1 out]
          }
          frame True {
          }
        }
        n509 = while {
          tunnel: [w1060] -> w949
          tunnel: [w1062] -> w961
          tunnel: w948 -> [w1058]
          tunnel: [w1058] -> w947
          stop <- w1063 stop-if-true
          n510 = local read "Zernike Enable"() -> (w1061:bool[])
          n511 = local read "Current Z Idx"() -> (w1059:i32)
          n512 = Index Array(array=w1061, index=w1059) -> (element=w1066:bool)
          n513 = Array Size(array=w1061) -> (size(s)=w1065:i32)
          n514 = case shown="False" w1066 {
            tunnel: w1059 -> [w1069 w1071]
            tunnel: [w1068 w1071] -> w1060
            tunnel: [FALSE ("2D Time-Lapse Measure") TRUE ("2D Time-Lapse Measure")] -> w1064
            frame False {
              n515 = Increment(x=w1069) -> (x+1=w1068:i32)
            }
            frame True {
            }
          }
          n516 = Greater Or Equal?(x=w1060, y=w1065) -> (x >= y?=w1062:bool)
          n517 = local write "Current Z Idx"(w1060) -> ()
          n518 = Compound Arithmetic op=OR(w1064, w1062) -> (w1063:bool)
        }
        n519 = local read "Stop AO Algorithm"() -> (w960:bool)
        n520 = Compound Arithmetic op=OR(w961, w960) -> (w962:bool)
        n521 = case shown="False" w962 {
          tunnel: w951 -> [w1017 _]
          tunnel: w956 -> [w1011 w1052]
          tunnel: w947 -> [w996 w1051]
          tunnel: w949 -> [w1010 _]
          tunnel: [w1003 w1051] -> w958
          tunnel: [w1001 w1052] -> w957
          frame False {
            w1002 = TRUE ("Value (Signaling)")
            n522 = Equal To 0?(x=w1017) -> (x = 0?=w1016:bool)
            n523 = case shown="False" w1016 {
              tunnel: [w1029 dbl[] [0.0, 0.0, 0.0, 0.0, 0.0, 0.0, 0.0, 0.0, 0.0, 0.0, 0.0, 0.0] ("Zernike Array")] -> w1007
              tunnel: w1010 -> [w1021 _]
              tunnel: [w1023 w1048] -> w998
              tunnel: [w1019 w1048] -> w994
              tunnel: w996 -> [w1020 w1046]
              tunnel: [w1020 w1045] -> w995
              frame False {
                n524 = local read "Zernike Array"() -> (w1031:dbl[])
                n525 = local read "Z Direction"() -> (w1027:bool)
                n526 = local read "Metric Value"() -> (w1024:dbl)
                n527 = Index Array(array=w1031, index=w1021) -> (element=w1030:dbl)
                n528 = case shown="True" w1027 {
                  tunnel: w1030 -> [_ w1036]
                  tunnel: [-1.0 w1038] -> w1025
                  tunnel: w1024 -> [_ w1037]
                  tunnel: [nan ("Metric Value") w1037] -> w1023
                  tunnel: [nan ("Z4: Ast45") w1036] -> w1019
                  frame False {
                    n529 = local write "Z Direction"(TRUE ("Zernike Dir")) -> ()
                  }
                  frame True {
                    n530 = Add(x=w1036, y="Z Cali Step") -> (x+y=w1038:dbl)
                  }
                }
                n531 = Greater?(x=w1025, y=1.0) -> (0:w1028:bool)
                n532 = case shown="True" w1028 {
                  tunnel: w1021 -> [_ w1043]
                  tunnel: w1025 -> [w1040 _]
                  tunnel: [w1040 0.0] -> w1022
                  frame False {
                  }
                  frame True {
                    n533 = Increment(x=w1043) -> (x+1=w1044:i32)
                    n534 = local write "Current Z Idx"(w1044) -> ()
                    n535 = local write "Z Direction"(FALSE ("Zernike Dir")) -> ()
                  }
                }
                n536 = Replace Array Subset(array=w1031, new element=w1022, index=w1021) -> (w1029:dbl[])
              }
              frame True {
                w1048 = nan ("Metric Value")
                n537 = local write "Z Direction"(FALSE ("Zernike Dir")) -> ()
                n538 = property on="Metric Calibration" class="WFChart (strict)"(error in=w1046, "History Data"=dbl[][] []) -> (error out=w1045:errorcluster)  [unwired: 1 in, 1 out]
              }
            }
            n539 = Increment(x=w1017) -> (x+1=w1018:sgl)
            n540 = local write "Current Iteration"(w1018) -> ()
            n541 = In Range and Coerce(upper limit=1.0 ("y"), x=w1007, lower limit=-1.0 ("y")) -> (coerced(x)=w1006:dbl[])  [unwired: 1 out]
            n542 = call "TLDFMX Calculate Zernike Pattern.vi"("error in (no error)"=w995, "Zernike Amplitudes"=w1006, "Zernikes"=u32 4294967295, "instrument handle"=w1011) -> ("error out"=w1012:errorcluster, "Mirror Pattern"=w1013:dbl[], "instrument handle out"=w1014:refnum<visa-resource-name>)  [unwired: 5 in]
            n543 = call "TLDFM Set Segment Voltages.vi"("error in (no error)"=w1012, "Segment Voltages"=w1013, "instrument handle"=w1014) -> ("error out"=w1005:errorcluster, "instrument handle out"=w1001:refnum<visa-resource-name>)  [unwired: 7 in]
            n544 = property on="Fast Scan" class="Bool (strict)"(error in=w1005, "Val(Sgnl)"=w1002) -> (error out=w1004:errorcluster)  [unwired: 1 in, 1 out]
            n545 = property on="Export Z Calibration" class="Bool (strict)"(error in=w1004, "Val(Sgnl)"=w1002) -> (error out=w1003:errorcluster)  [unwired: 1 in, 1 out]
            n546 = Build Array(w994) -> (w999:dbl[])
            n547 = Build Array(w998) -> (w997:dbl[])
            n548 = local write "Zernike Array"(w1006) -> ()
            n549 = Build Array(w999, w997) -> (→"Metric Calibration":dbl[][])
          }
          frame True {
            w1053 = FALSE ("2D Time-Lapse Measure")
            n550 = local write "Export Z Calibration"(w1053) -> ()
            n551 = local write "Current Iteration"(sgl 0.0 ("Current Step")) -> ()
            n552 = local write "Z Direction"(FALSE ("Zernike Dir")) -> ()
            n553 = local write "Fast Scan Progress"(0.0 ("Fast Scan Progress")) -> ()
            n554 = local write "Current Z Idx"(0 ("Curr Zernike Idx")) -> ()
            n555 = local write "Fast Scan"(w1053) -> ()
            n556 = local write "Stop Fast Scan"(w1053) -> ()
            n557 = local write "Stop AO Algorithm"(w1053) -> ()
          }
        }
      }
      event "Measure": Value Change {
        n558 = event-data() -> ()  [unwired: 1 in, 1 out]
        n559 = flat-sequence {
          tunnel: w1094 -> [w1099]
          tunnel: [w1099] -> w1093
          tunnel: [w1098] -> w1091
          tunnel: [w1097] -> w1089
          tunnel: w1088 -> [w1097]
          tunnel: [w1096] -> w1087
          tunnel: w1086 -> [w1096]
          tunnel: w1083 -> [w1095]
          tunnel: [w1095] -> w1082
          tunnel: w1093 -> [w1132]
          tunnel: [w1132] -> w1092
          tunnel: w1091 -> [w1107]
          tunnel: [w1107] -> w1090
          tunnel: w1089 -> [w1129]
          tunnel: w1087 -> [w1125]
          tunnel: [w1124] -> w1084
          tunnel: w1082 -> [w1119]
          tunnel: [w1112] -> w1078
          tunnel: [w1106] -> w1076
          tunnel: [w1103] -> w1075
          tunnel: [w1102] -> w1074
          tunnel: w1092 -> [w1199]
          tunnel: w1090 -> [w1198]
          tunnel: w1084 -> [w1196]
          tunnel: [w1199] -> w1081
          tunnel: [w1192] -> w1080
          tunnel: w1078 -> [w1197]
          tunnel: [w1198] -> w1077
          tunnel: w1076 -> [w1195]
          tunnel: w1075 -> [w1194]
          tunnel: w1074 -> [w1193]
          tunnel: [w1253] -> w1085
          tunnel: [w1255] -> w1079
          tunnel: w1081 -> [w1255]
          tunnel: w1080 -> [w1253]
          tunnel: w1077 -> [w1249]
          frame #0 {
            n560 = Tick Count (ms)() -> (millisecond timer value=w1098:u32)
          }
          frame #1 {
            w1130 = T13."Measurement" ("Main Tab")
            n561 = local read "Calibrated Bias (V)"() -> (w1113:dbl[])
            n562 = call "ScanXY.vi"("Scan/Meas Parameters"="Measurement Parameters") -> ("XYcoordinates"=w1116:dbl[][])  [unwired: 10 in]
            n563 = Unbundle By Name("Measurement Parameters") -> ("Pixel Size"=w1122:dbl)
            n564 = case shown="True" "Single Pixel Measure?" {
              tunnel: [w1133 w1134] -> w1115
              tunnel: w1116 -> [w1133 w1135]
              frame False {
              }
              frame True {
                n565 = Multiply(x=w1135, y=0.0) -> (x*y=w1134:dbl[][])
              }
            }
            n566 = call "DAQInit.vi"("Scan/Meas Parameters"="Measurement Parameters", "error in"=w1119, "Functions"=w1130, "Global Parameters"=w1125, "DAQ Channels"=w1129) -> ("error out"=w1120:errorcluster, "Expected Time (s)"=→"Expected Frame Time (s)":dbl, "Tasks Out"=w1131:T14)  [unwired: 4 in]
            n567 = To Long Integer(number=w1122) -> (32bit integer=w1121:i32)
            n568 = while {
              tunnel: w1131 -> [w1184]
              tunnel: w1130 -> [w1153]
              tunnel: w1120 -> [w1143]
              tunnel: w1115 -> [w1183]
              tunnel: w1113 -> [w1182]
              tunnel: w1125 -> [w1151]
              tunnel: "Measurement Parameters" -> [w1152]
              tunnel: [w1180] -> w1128
              tunnel: [w1153] -> w1127
              tunnel: [w1147] -> w1126
              tunnel: [w1158] -> w1124
              tunnel: w1121 -> [w1158]
              tunnel: "# of Frames to Average" -> [w1171]
              tunnel: [w1141] -> w1111
              tunnel: [w1140] -> w1110
              tunnel: [w1139] -> w1109
              tunnel: [w1138] -> w1108
              tunnel: [w1137] -> w1106
              i -> [w1169]
              stop <- w1178 stop-if-true
              n569 = local read "Shutter"() -> (w1144:bool)
              n570 = To Unsigned Long Integer(number=w1169) -> (unsigned 32bit integer=w1157:u32)